vi "neuKLEIN.vi"() -> ()   [LabVIEW 2016] (continued)
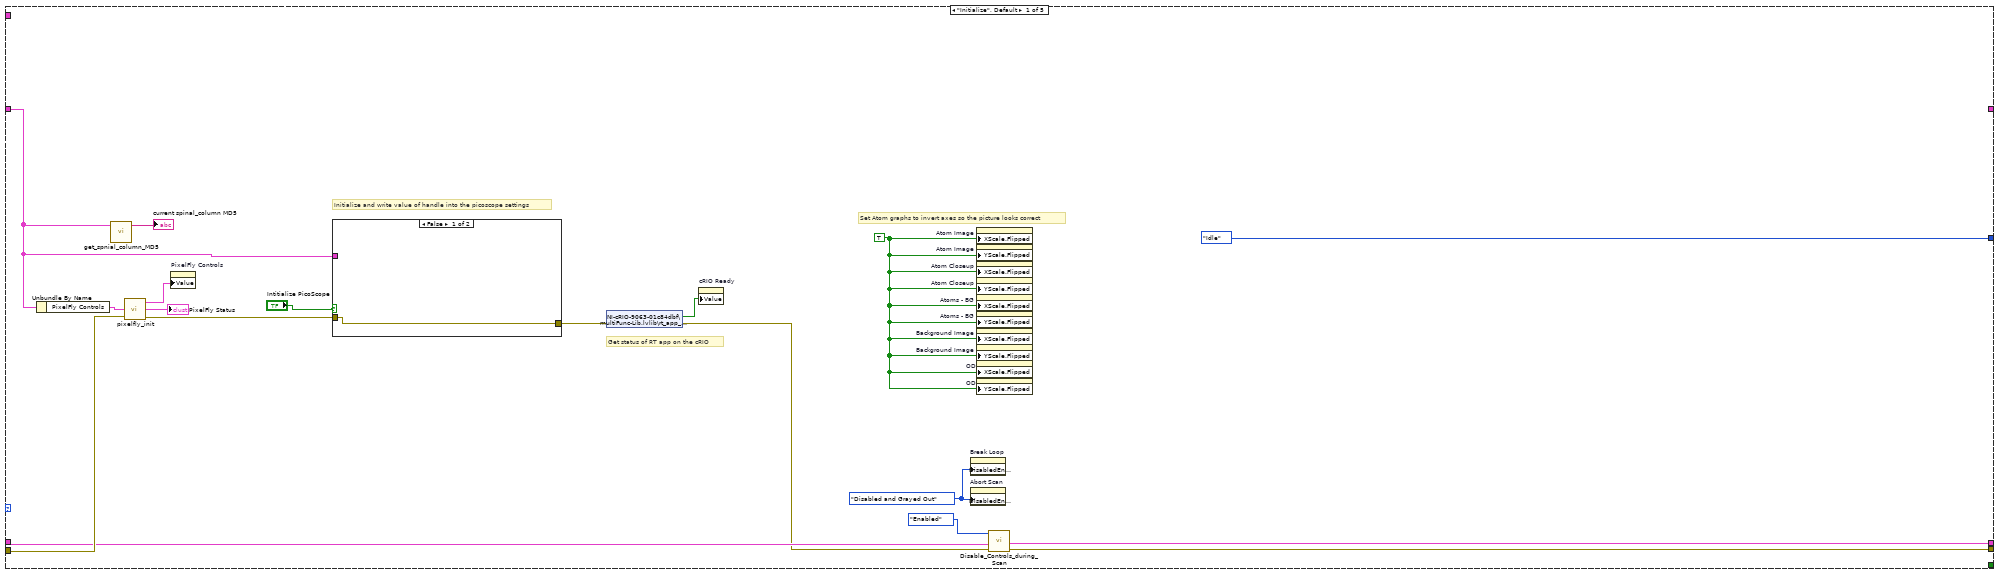
[diagram p2: hidden frame]
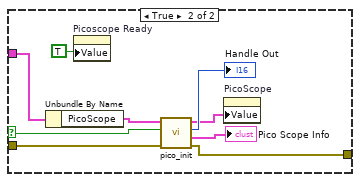
[diagram p3: hidden frame]
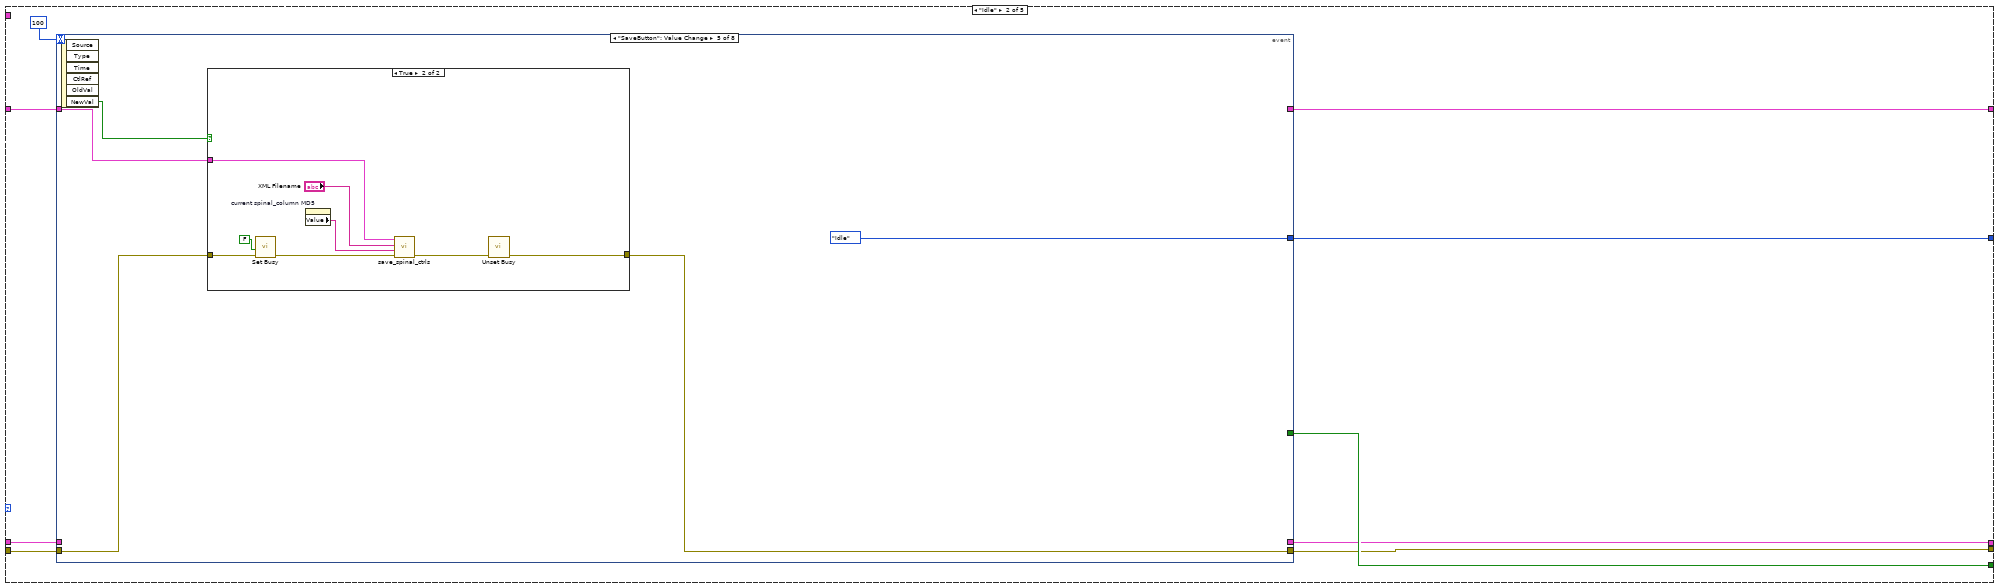
[diagram p4: hidden frame]
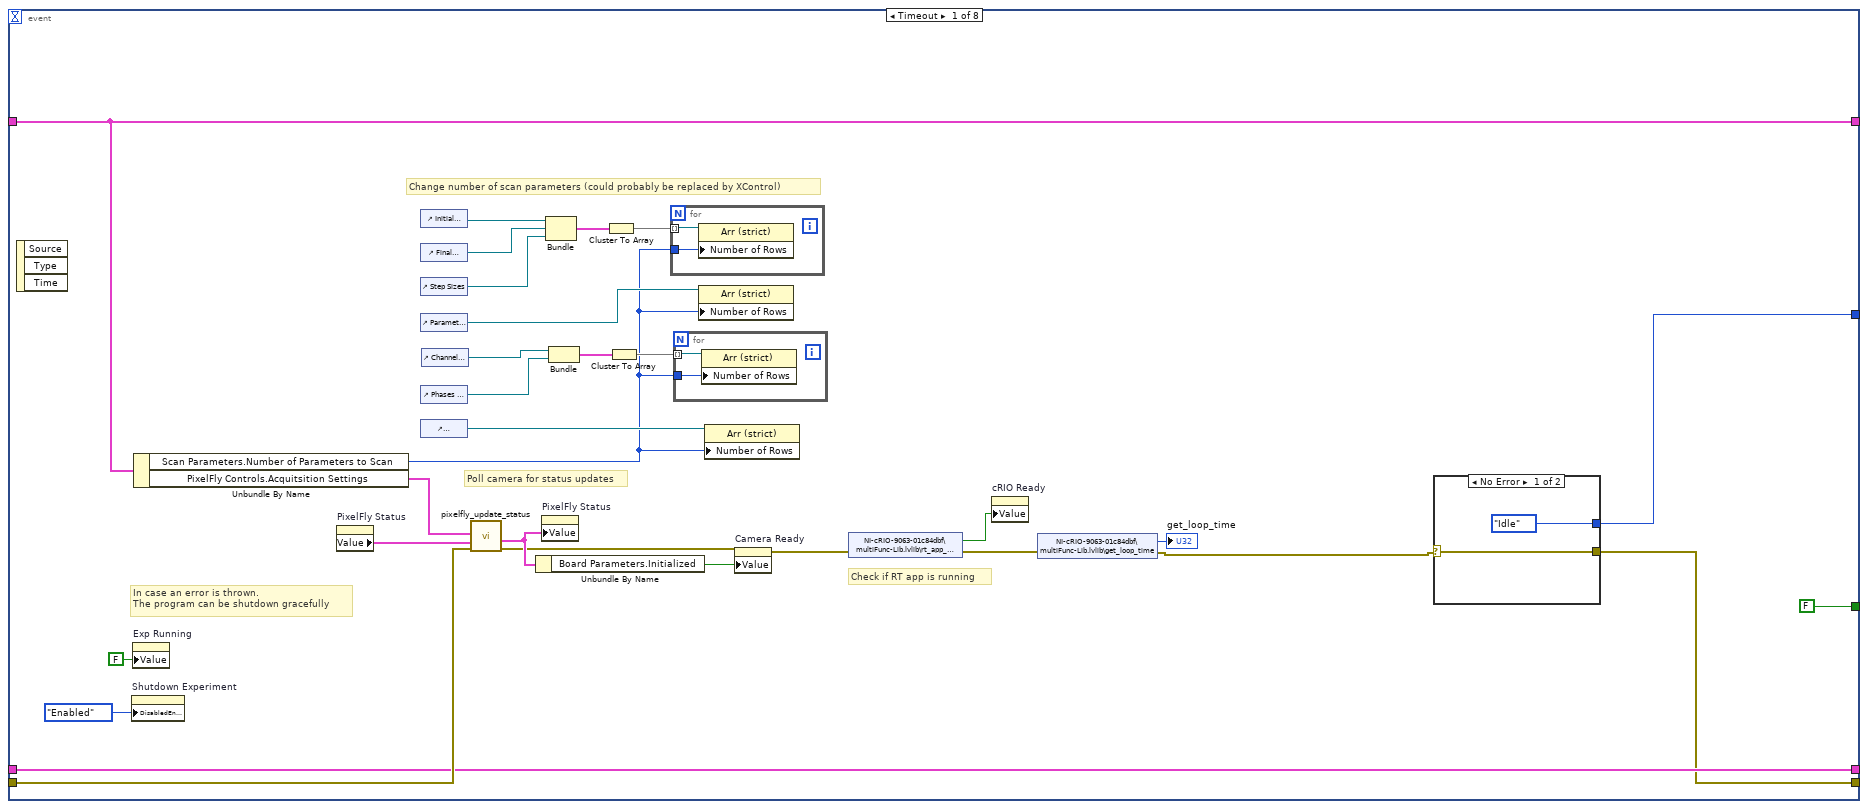
[diagram p5: hidden frame]
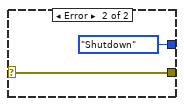
[diagram p6: hidden frame]
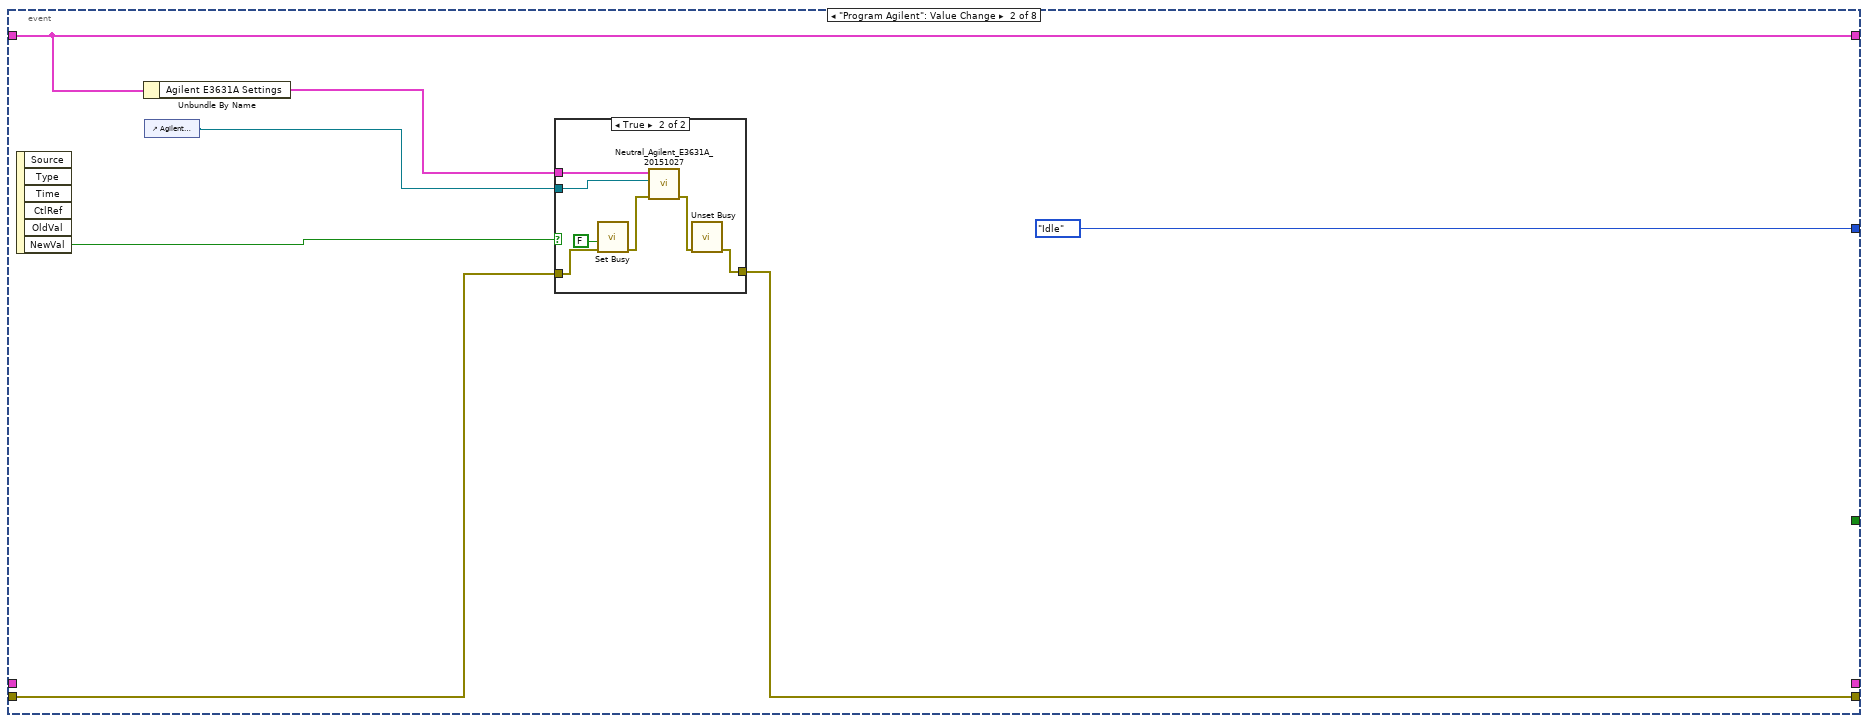
[diagram p7: hidden frame]
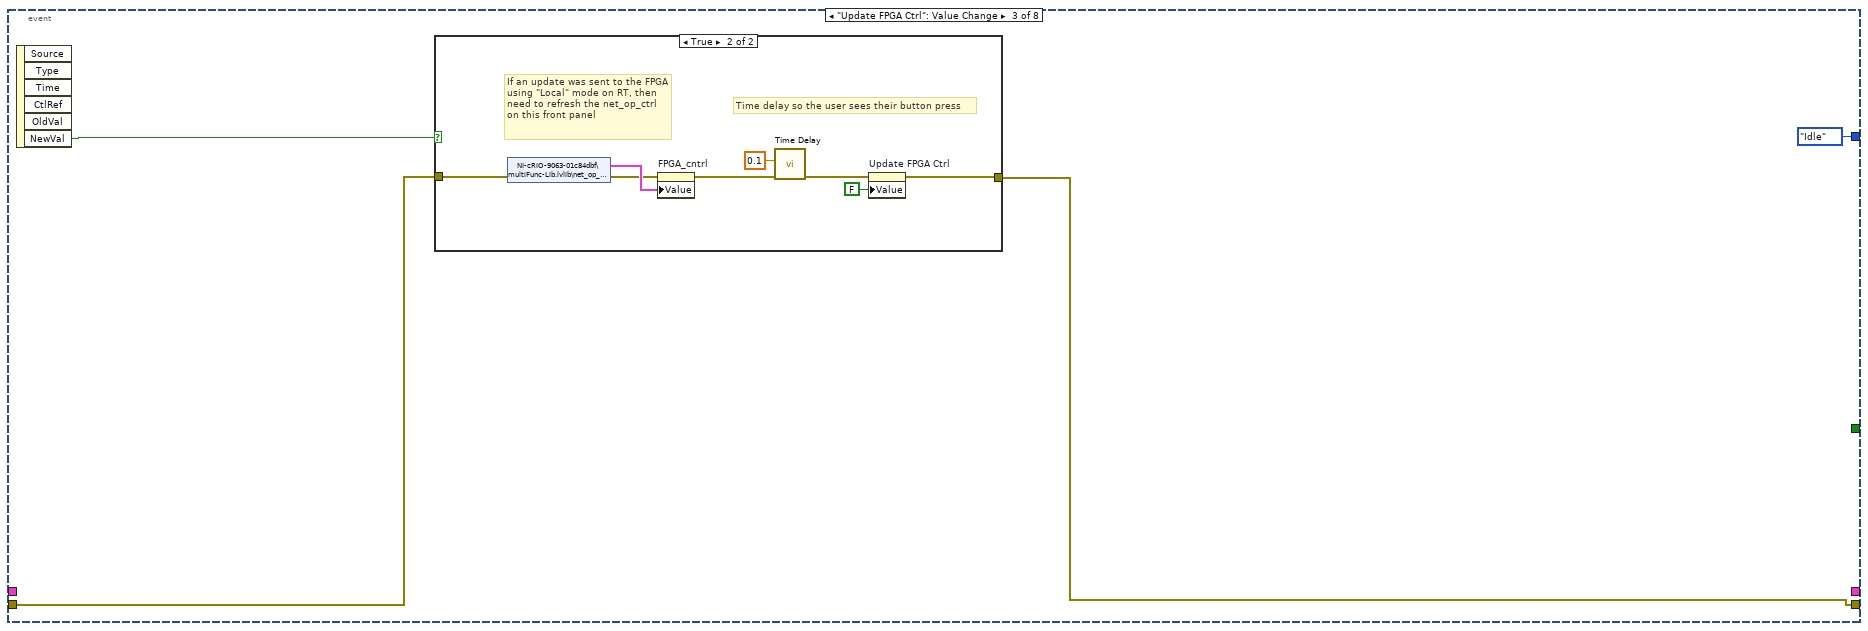
[diagram p9: hidden frame]
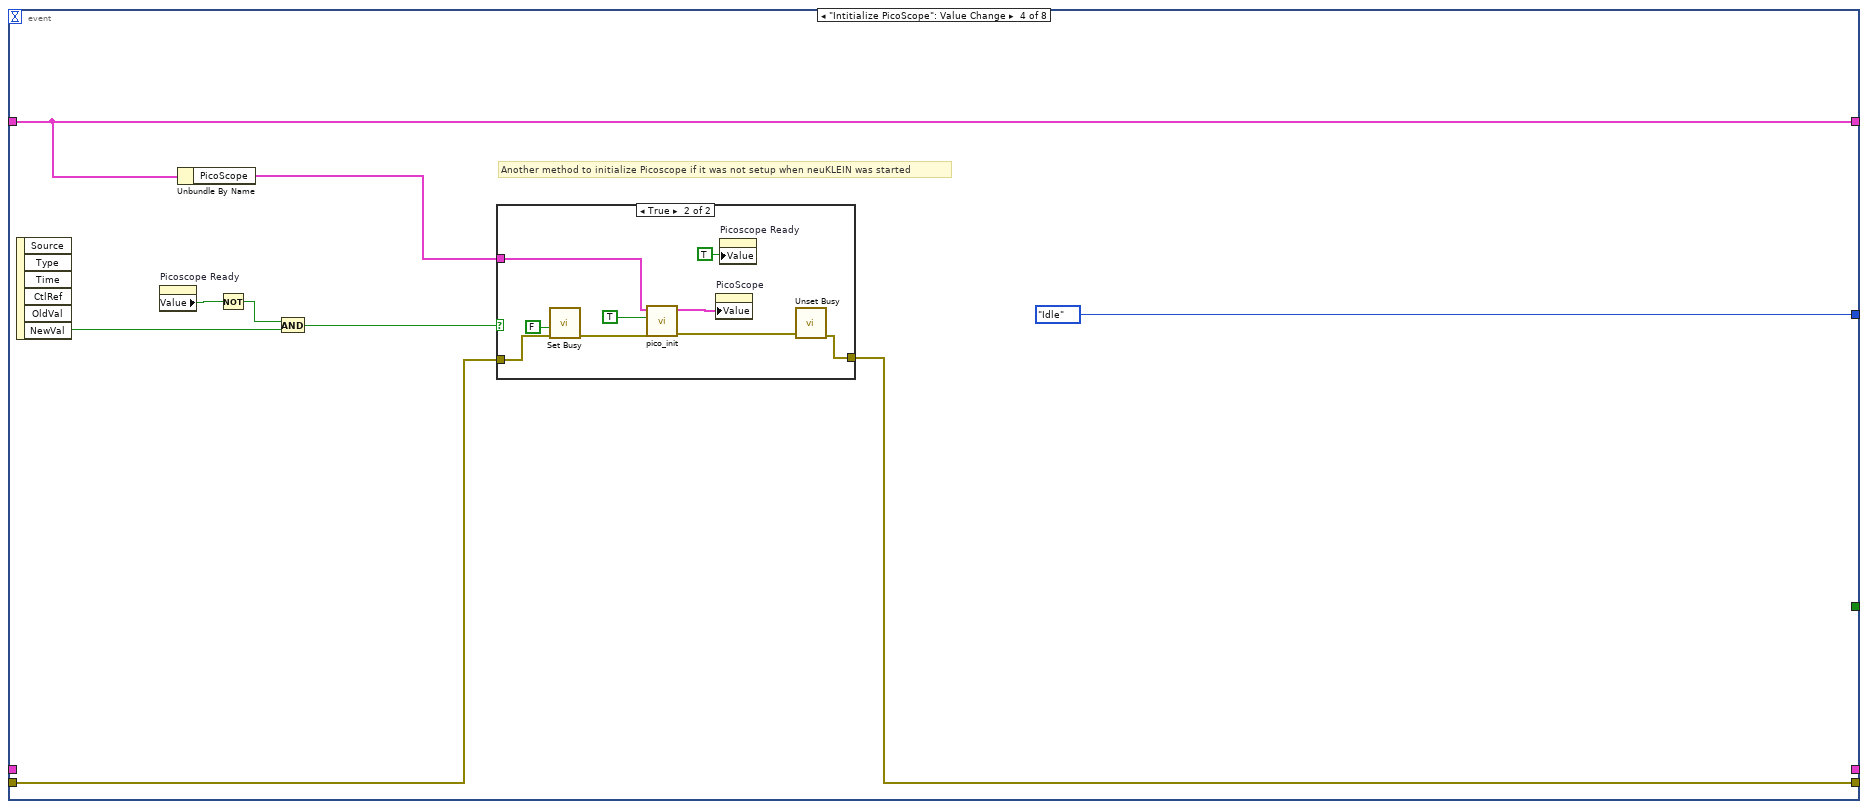
[diagram p11: hidden frame]
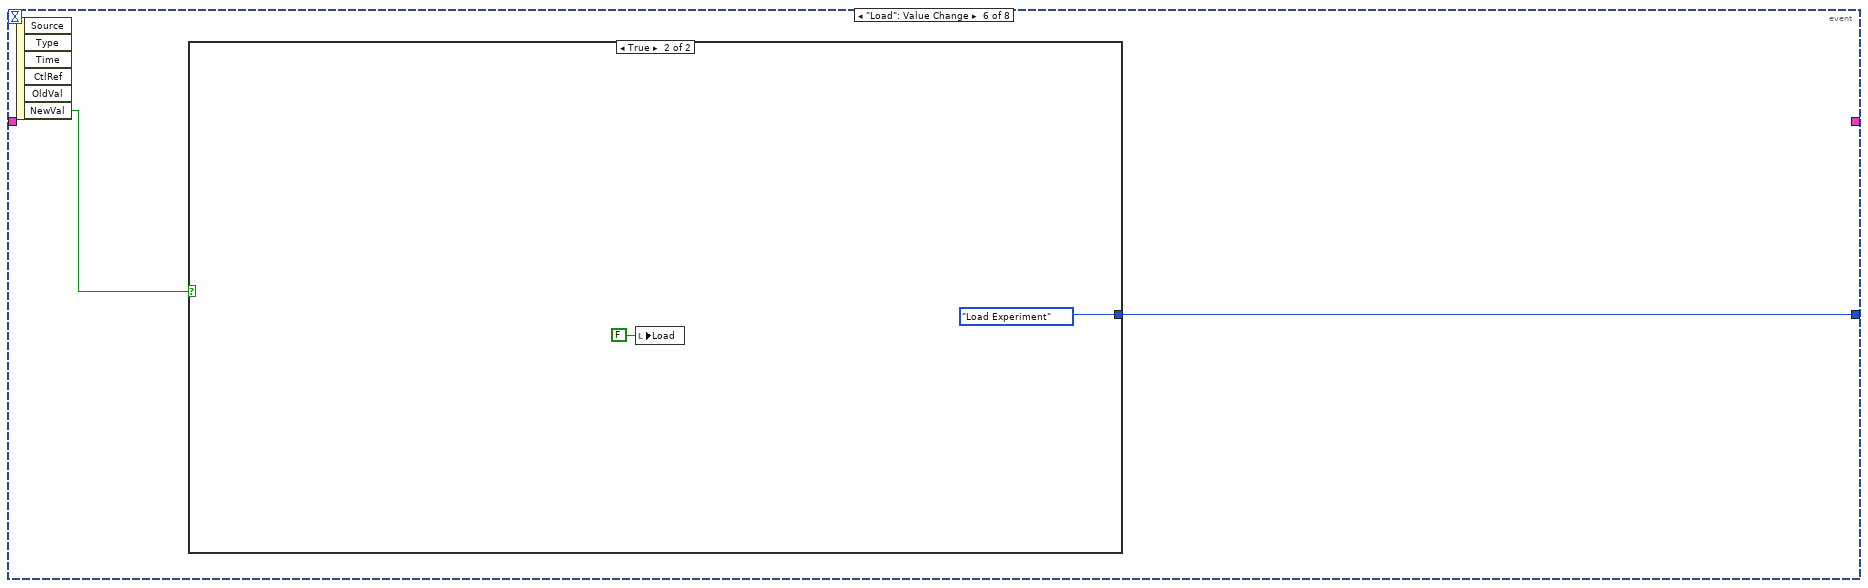
[diagram p14: hidden frame]
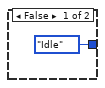
[diagram p15: hidden frame]
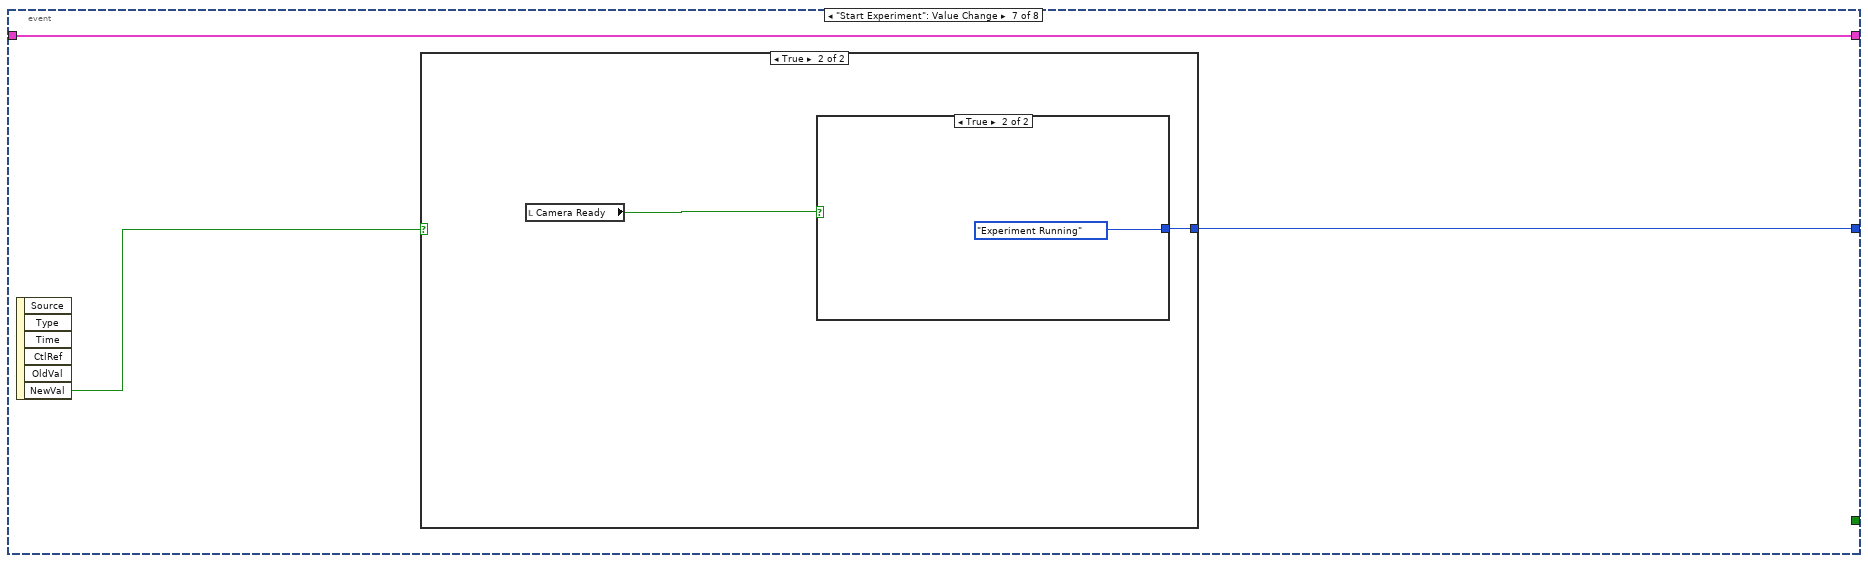
[diagram p16: hidden frame]
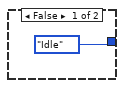
[diagram p17: hidden frame]
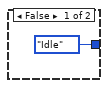
[diagram p18: hidden frame]
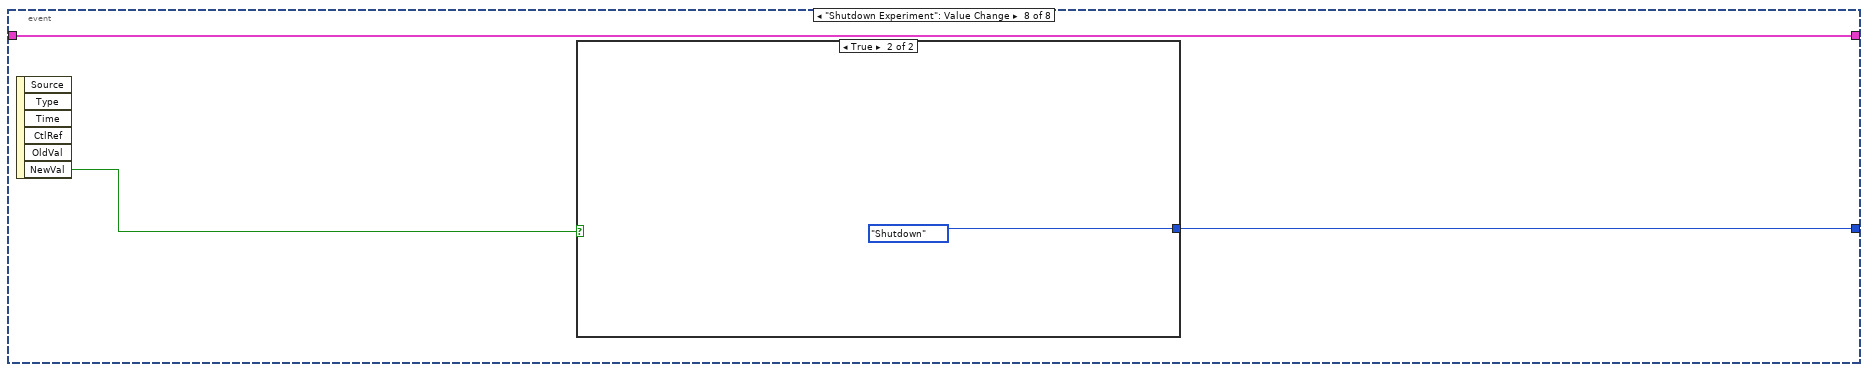
[diagram p19: hidden frame]
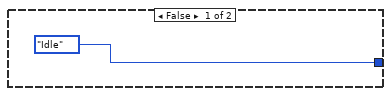
[diagram p20: hidden frame]
              frame False {
              }
              frame True {
                n79 = call <vilib>:"Set Busy.vi"("error in (no error)"=w147, "disable click? (T)"=FALSE) -> ("error out"=w144:errorcluster)  [unwired: 8 in, 1 out]
                n80 = call "pico_init.vi"("error in (no error)"=w144, "Initialize PicoScope?"=TRUE, "PicoScope Acquisition Settings Input"=w142) -> ("error out"=w143:errorcluster, "PicoScope Acquisition Settings Output"=w140:T39)  [unwired: 4 in, 2 out]
                n81 = property on="PicoScope" class="Clust (strict)"("Value"=w140) -> ()  [unwired: 2 in, 2 out]
                n82 = property on="Picoscope Ready" class="Bool (strict)"("Value"=TRUE ("Picoscope Ready")) -> ()  [unwired: 2 in, 2 out]
                n83 = call <vilib>:"Unset Busy.vi"("error in (no error)"=w143) -> ("error out"=w146:errorcluster)  [unwired: 10 in]
              }
            }
          }
          event "SaveButton": Value Change {
            n84 = event-data() -> ("NewVal"=w152:bool)  [unwired: 1 in, 5 out]
            n85 = case shown="True" w152 {
              tunnel: w151 -> [_ w156]
              tunnel: w149 -> [w153 w160]
              tunnel: [w153 w159] -> w148
              frame False {
              }
              frame True {
                n86 = call <vilib>:"Set Busy.vi"("error in (no error)"=w160, "disable click? (T)"=FALSE) -> ("error out"=w158:errorcluster)  [unwired: 8 in, 1 out]
                n87 = property on="current spinal_column MD5" class="Str"() -> ("Value"=w154:string)  [unwired: 2 in, 2 out]
                n88 = call "save_spinal_ctrls.vi"("error in (no error)"=w158, "MD5"=w154, "Name for file"="XML Filename", "spinal_column"=w156) -> ("error out"=w157:errorcluster)  [unwired: 5 in, 2 out]
                n89 = call <vilib>:"Unset Busy.vi"("error in (no error)"=w157) -> ("error out"=w159:errorcluster)  [unwired: 10 in]
              }
            }
          }
          event "Load": Value Change {
            n90 = event-data() -> ("NewVal"=w163:bool)  [unwired: 1 in, 5 out]
            n91 = case shown="True" w163 {
              tunnel: [rydberg_state_machine_states."Idle" rydberg_state_machine_states."Load Experiment"] -> w162
              frame False {
              }
              frame True {
                n92 = local write "Load"(FALSE ("Load")) -> ()
              }
            }
          }
          event "Start Experiment": Value Change {
            n93 = event-data() -> ("NewVal"=w169:bool)  [unwired: 1 in, 5 out]
            n94 = case shown="True" w169 {
              tunnel: [rydberg_state_machine_states."Idle" w172] -> w168
              frame False {
              }
              frame True {
                n95 = local read "Camera Ready"() -> (w171:bool)
                n96 = case shown="True" w171 {
                  tunnel: [rydberg_state_machine_states."Idle" rydberg_state_machine_states."Experiment Running"] -> w172
                  frame False {
                  }
                  frame True {
                  }
                }
              }
            }
          }
          event "Shutdown Experiment": Value Change {
            n97 = event-data() -> ("NewVal"=w177:bool)  [unwired: 1 in, 5 out]
            n98 = case shown="True" w177 {
              tunnel: [rydberg_state_machine_states."Idle" rydberg_state_machine_states."Shutdown"] -> w176
              frame False {
              }
              frame True {
              }
            }
          }
        }
      }
      frame "Experiment Running" {
        w180 = T62 3 items=["no dialog", "OK message", "continue or stop message", "OK message + warnings", "continue/stop + warnings"] ("type of dialog (OK msg:1)")
        # "Open Atom Shutter"
        # "Continue Exp. Running state if not aborted,\nno error, and Trigger Snap true"
        n99 = Unbundle By Name(w188) -> ("Scan Parameters"=w187:T5)
        n100 = property on="Trigger Snap Mode" class="Bool (strict)"() -> ("Value"=w190:bool)  [unwired: 2 in, 2 out]
        n101 = Get Date/Time In Seconds() -> (seconds since 1Jan1904=w204:timestamp)
        n102 = local write "Exp Running"(TRUE) -> ()
        n103 = local write "Start Experiment"(FALSE ("Start Experiment")) -> ()
        n104 = call "calculate_parameters.vi"("Experimental Variables"=w196) -> ("Calculated Experimental Values"=→"Calculated Experimental Values":T10)  [unwired: 8 in, 2 out]
        n105 = call "Disable_Controls_during_Scan.vi"("Error In"=w203, "Control Reference Cluster Input"=w191, "Control State In"=T58."Disabled and Grayed Out" ("Disabled")) -> ("error out"=w194:errorcluster, "Control Reference Cluster Output"=w201:T56)  [unwired: 7 in]
        n106 = property on="Abort Scan" class="Bool (strict)"("DisabledEnum"=T58."Enabled" ("Disabled")) -> ()  [unwired: 2 in, 2 out]
        n107 = call "GenerateScanArrays.vi"("time stamp"=w204, "In Trigger Snap Mode?"=w190, "Scan Parameters"=w187) -> ("Parameter Array"=w192:dbl[][], "Array"=w195:dbl[])  [unwired: 6 in, 1 out]
        n108 = call "Progress Bar Initialization.vi"("Array"=w192, "Trigger Snap or Scan?"=w190, "error in (no error)"=w194) -> ("Scan Progress"=w186:T49, "error out"=w193:errorcluster)  [unwired: 6 in]
        n109 = call "atomShutterCtrl.vi"("Atom Shutter"=TRUE) -> ()
        n110 = property on="Scan Progress" class="Clust (strict)"("Value"=w186) -> ()  [unwired: 2 in, 2 out]
        n111 = for {
          tunnel: w190 -> [w258]
          shift-right: [w232] -> _
          shift-left: w188 -> [w231]
          shift-right: [w238] -> w185
          shift-left: w193 -> [w271]
          tunnel: w192 -> [w260] mode=indexing
          tunnel: w195 -> [w255]
          tunnel: w204 -> [w253]
          tunnel: w201 -> [w245]
          tunnel: [w245] -> w200
          tunnel: w196 -> [w247]
          tunnel: ["Abort Scan"] -> w183
          i -> [w246]
          stop <- "Abort Scan" stop-if-true
          # "This is going to execute at the beginning of the loop.\nWill try to fix it when I get aruond to implementing a\nfull state machine"
          # "Allows for scans to be aborted"
          n112 = call "Change_ParameterV2.vi"("Started In Trig Snap?"=w258, "Parameter Values In"=w260, "Spinal Column In"=w231) -> ("Current Parameter Values"=w254:dbl[], "Spinal Column Out"=w259:T63)  [unwired: 7 in]
          "Current Param. Values" <- w254
          n113 = property on="Take Pictures" class="Bool (strict)"() -> ("Value"=w234:bool)  [unwired: 2 in, 2 out]
          n114 = call "WriteExp.vi"("error in (no error)"=w271, "Take Pictures"=w234, "Spinal Column In"=w259) -> ("error out"=w249:errorcluster, "Spinal Column Out"=w263:T63)  [unwired: 7 in]
          n115 = call "DoExperiment.vi"("Spinal Column In"=w263, "Take Pictures"=w234, "Error In"=w249) -> ("error out"=w238:errorcluster, "Channel B Out"=w243:dbl[][][], "Channel A Out"=w242:dbl[][][], "Spinal Column Out"=w250:T63, "Atom Image"=w270:dbl[][], "Background Image"=w269:dbl[][], "Buffer status"=→"Buffer status":T14, "Wavemeter"=w233:string)  [unwired: 9 in]
          "Wavemeter" <- w233
          n116 = call "rapid_xy.vi"("Channel A Out"=w242) -> ("xy array"=→"Pico Scope Channel A":T53)  [unwired: 10 in]
          n117 = call "rapid_xy.vi"("Channel A Out"=w243) -> ("xy array"=→"Pico Scope Channel B":T53)  [unwired: 10 in]
          n118 = call "BG_Subtraction.vi"("Background Image"=w269, "Atom Image"=w270) -> ("Background Image Out"=w257:dbl[][], "Atom Image Out"=w265:dbl[][], "Atoms - BG"=w266:dbl[][])  [unwired: 7 in]
          "Atom Image" <- w265
          "Background Image" <- w257
          "Atoms - BG" <- w266
          n119 = property on="Atoms - BG" class="IntGraph (strict)"() -> ("CrsrLis"=w267:T64)  [unwired: 2 in, 2 out]
          n120 = call "CutIMG.vi"("Full Image In"=w266, "Cursor List"=w267) -> ("Cut Image Out"=→"Atom Closeup":dbl[][])  [unwired: 9 in]
          n121 = case shown="\"Fancy\"" "Set Analysis Mode" {
            tunnel: w267 -> [w282 w296]
            tunnel: w265 -> [w281 w295]
            tunnel: w257 -> [w280 w294]
            tunnel: [w279 w293] -> w256
            tunnel: [w278 w291] -> w228
            tunnel: [w273 w290] -> w241
            tunnel: [w276 w289] -> w236
            tunnel: [w276 w288] -> w235
            tunnel: w247 -> [w277 w287]
            tunnel: [T52 {"Amplitude (OD)"=0.0, "X Center (px)"=0.0, "Y Center (px)"=0.0, " X Width (um)"=0.0, "Y Width (um)"=0.0, "Aspect Ratio"=0.0, "Rot. Angle (deg)"=0.0} ("Best Fit Parameter Cluster") w286] -> w240
            tunnel: [u32 0 ("Elapsed time ( ms)") w285] -> w239
            tunnel: [0.0 ("Phase Space Density") w284] -> w237
            frame "Fast", Default {
              w276 = 1.0 ("Temperature (K) x")
              n122 = call "CountAtomsFast.vi"("Experimental Variables"=w277, "Background Image"=w280, "Atom Image"=w281, "Cursor List"=w282) -> ("Data Cuts"=w273:dbl[][], "OD"=w279:dbl[][], "Number"=w278:dbl)  [unwired: 5 in]
            }
            frame "Fancy" {
              n123 = call "CountAtoms_LVFitting.vi"("Cursor List"=w296, "Atom Image"=w295, "Experimental Variables"=w287, "Background Image"=w294, "Drop Time"="Drop Time", "Trap Frequencies"="Trap Frequencies") -> ("Elapsed time ( ms)"=w285:u32, "Number"=w291:dbl, "OD"=w293:dbl[][], "Data Cuts"=w290:dbl[][], "Temperature (K) x"=w289:dbl, "Phase Space Density"=w284:dbl, "Best Fit Parameter Cluster"=w286:T52, "Temperature (K) y"=w288:dbl)  [unwired: 1 in, 1 out]
            }
          }
          "GIANT Atoms" <- w256
          "OD" <- w256
          "Number" <- w228
          "Atom Number Chart" <- w228
          "Temp. (K) - Y" <- w235
          "Temp. (K) - X" <- w236
          "Giant Data Cuts" <- w241
          "Data Cuts" <- w241
          "Best Fit Parameter Cluster" <- w240
          "Elapsed time ( ms)" <- w239
          "Phase Space Density" <- w237
          n124 = property on="Atom Number Chart" class="WFChart (strict)"() -> ("XScale.Maximum"=w225:dbl)  [unwired: 2 in, 2 out]
          n125 = property on="Atom Number Chart" class="WFChart (strict)"() -> ("History Data"=w224:dbl[])  [unwired: 2 in, 2 out]
          n126 = property on="Temperature Chart" class="WFChart (strict)"() -> ("History Data"=w223:T65)  [unwired: 2 in, 2 out]
          n127 = Bundle("Temperature (K) x"=w236, "Temperature (K) y"=w235) -> (→"Temperature Chart":T51)  [unwired: 1 in]
          n128 = Bundle(cluster="output cluster", "Number"=w228, "OD"=w256, "Data Cuts"=w241, "Temperature (K) x"=w236, "Temperature (K) y"=w235) -> (w252:T46)
          n129 = case shown="False" w258 {
            tunnel: w270 -> [w312 _]
            tunnel: w269 -> [w311 _]
            tunnel: w243 -> [w310 _]
            tunnel: w242 -> [w309 _]
            tunnel: w255 -> [w308 _]
            tunnel: w246 -> [w299 _]
            tunnel: w254 -> [w307 _]
            tunnel: w253 -> [w306 _]
            tunnel: w250 -> [w305 w313]
            tunnel: w252 -> [w304 _]
            tunnel: [w300 w313] -> w232
            tunnel: w233 -> [w297 _]
            frame False {
              # "Increment progress bar"
              n130 = Increment(x=w299) -> (x+1=w298:i32)
              n131 = property on="Current Pnt Num" class="DigNum (strict)"("Value"=w298) -> ()  [unwired: 2 in, 2 out]
              n132 = call "GenerateBatchFilesV2.vi"("Spinal Column In"=w305, "output cluster"=w304, "time stamp"=w306, "Current Values"=w307, "Loop Iteration"=w299, "Wavemeter"=w297, "Independent Variable Array"=w308) -> ("Scan Parameters.Raw_Data Folder"=w303:path, "Spinal Column Out"=w300:T63, "Full Scan Name Out"=w301:string, "Image Number"=w302:i32)  [unwired: 3 in, 2 out]
              "Scan Name" <- w301
              n133 = call "SaveImages.vi"("Background Image In"=w311, "Atoms Image In"=w312, "Base Filename"=w301, "Raw Data Path"=w303, "ImageNumber"=w302) -> ()  [unwired: 9 in, 2 out]
              n134 = call "save_pico_data.vi"("full scan name"=w301, "Img #"=w302, "Channel B In"=w310, "Channel A In"=w309, "Spinal Column In"=w300) -> ()  [unwired: 7 in]
            }
            frame True {
            }
          }
          n135 = Bundle("XScale.Maximum"=w225, "History Data"=w224, "History Data"=w223) -> (w222:T66)  [unwired: 1 in]
          n136 = call "numAndTempStats.vi"("Stat. Limits"="Stat. Limits", "Stats Flag"="Stats Flag", "strip chart properties"=w222) -> ("Num and Temp Stats"=→"Num and Temp Stats":T47)  [unwired: 8 in]
        }
        n137 = property on="Trigger Snap Mode" class="Bool (strict)"() -> ("Value"=w184:bool)  [unwired: 2 in, 2 out]
        n138 = Compound Arithmetic op=AND(invert w183, w184, invert w185) -> (w182:bool)
        n139 = case shown="False" w182 {
          tunnel: [rydberg_state_machine_states."Idle" rydberg_state_machine_states."Experiment Running"] -> w207
          tunnel: w185 -> [w215 w219]
          tunnel: [w214 w219] -> w181
          tunnel: w200 -> [w212 w220]
          tunnel: [w211 w220] -> w199
          frame False {
            # "Close Atom Shutter"
            # "Reset abort button if pressed"
            n140 = property on="Abort Scan" class="Bool (strict)"() -> ("Value"=w210:bool)  [unwired: 2 in, 2 out]
            n141 = case shown="True" w210 {
              frame False {
              }
              frame True {
                # "Reset this in case it is true"
                n142 = property on="Abort Scan" class="Bool (strict)"("Value"=FALSE) -> ()  [unwired: 2 in, 2 out]
                n143 = property on="Trigger Snap Mode" class="Bool (strict)"("Value"=FALSE ("Trigger Snap Mode")) -> ()  [unwired: 2 in, 2 out]
              }
            }
            n144 = property on="Abort Scan" class="Bool (strict)"("DisabledEnum"=T58."Disabled and Grayed Out" ("Disabled")) -> ()  [unwired: 2 in, 2 out]
            n145 = call "atomShutterCtrl.vi"("Atom Shutter"=FALSE) -> ()
            n146 = call "Disable_Controls_during_Scan.vi"("Error In"=w215, "Control Reference Cluster Input"=w212, "Control State In"=T58."Enabled" ("Disabled")) -> ("error out"=w214:errorcluster, "Control Reference Cluster Output"=w211:T56)  [unwired: 7 in]
          }
          frame True {
          }
        }
        n147 = call <vilib>:"Simple Error Handler.vi"("type of dialog (OK msg:1)"=w180, "error in (no error)"=w181) -> ()  [unwired: 3 in, 5 out]
      }
      frame "Load Experiment" {
        n148 = property on="current spinal_column MD5" class="Str"() -> ("Value"=w314:string)  [unwired: 2 in, 2 out]
        n149 = call <vilib>:"Set Busy.vi"("error in (no error)"=w323, "disable click? (T)"=FALSE) -> ("error out"=w317:errorcluster)  [unwired: 8 in, 1 out]
        n150 = call "load_spinal_ctrls.vi"("spinal_column"=w316, "MD5"=w314, "DAT File Location"="XML File Location", "error in (no error)"=w317) -> ("Spinal Column Out"=w319:T63, "error out"=w318:errorcluster)  [unwired: 4 in]
        n151 = call <vilib>:"Unset Busy.vi"("error in (no error)"=w318) -> ("error out"=w322:errorcluster)  [unwired: 10 in]
        n152 = Unbundle By Name(w319) -> ("48ch_pb_array"=w321:T3, "Red MOT 87 Inputs"=w335:T21, "ODT Params"=w333:T25, "Red MOT 88 Inputs"=w332:T21, "Agilent E3631A Settings"=w327:T43, "Scan Parameters"=w331:T5, "PicoScope"=w330:T39, "6713 Blue MOT"=w329:T16, "6229 Green Lattice Inputs"=w328:T28, "Novatech Synth Settings"=w325:T36[][], "FPGA_cntrl"=w320:T30)
        n153 = property on="48ch_pb_array" class="Arr (strict)"("Value"=w321) -> ()  [unwired: 2 in, 2 out]
        n154 = property on="Red MOT 87 Inputs" class="Clust (strict)"("Value"=w335) -> ()  [unwired: 2 in, 2 out]
        n155 = property on="ODT Params" class="Clust (strict)"("Value"=w333) -> ()  [unwired: 2 in, 2 out]
        n156 = property on="Red MOT 88 Inputs" class="Clust (strict)"("Value"=w332) -> ()  [unwired: 2 in, 2 out]
        n157 = property on="Agilent E3631A Settings" class="Clust (strict)"("Value"=w327) -> ()  [unwired: 2 in, 2 out]
        n158 = property on="Scan Parameters" class="Clust (strict)"("Value"=w331) -> ()  [unwired: 2 in, 2 out]
        n159 = property on="PicoScope" class="Clust (strict)"("Value"=w330) -> ()  [unwired: 2 in, 2 out]
        n160 = property on="6713 Blue MOT" class="Clust (strict)"("Value"=w329) -> ()  [unwired: 2 in, 2 out]
        n161 = property on="6229 Green Lattice Inputs" class="Clust (strict)"("Value"=w328) -> ()  [unwired: 2 in, 2 out]
        n162 = property on="Novatech Synth Settings" class="Arr (strict)"("Value"=w325) -> ()  [unwired: 2 in, 2 out]
        n163 = property on="FPGA_cntrl" class="Clust (strict)"("Value"=w320) -> ()  [unwired: 2 in, 2 out]
      }
      frame "Shutdown" {
        w336 = FALSE ("Value")
        # "Close Atom Shutter\nJust in case"
        n164 = call "atomShutterCtrl.vi"("Atom Shutter"=FALSE) -> ()
        n165 = local write "Shutdown Experiment"(FALSE ("Shutdown Experiment")) -> ()
        n166 = property on="Initialized" class="Bool (strict)"(error in=w344, "Value"=w336) -> (error out=w342:errorcluster)  [unwired: 1 in, 1 out]
        n167 = property on="Running" class="Bool (strict)"(error in=w342, "Value"=w336) -> (error out=w341:errorcluster)  [unwired: 1 in, 1 out]
        n168 = Unbundle By Name(w348) -> ("PicoScope.Pico Scope Inititalization Settings.Handle"=w347:i16, "PixelFly Controls.Acquitsition Settings"=w346:T12)
        n169 = property on="Camera Ready" class="Bool (strict)"(error in=w341, "Value"=w336) -> (error out=w340:errorcluster)  [unwired: 1 in, 1 out]
        n170 = property on="Picoscope Ready" class="Bool (strict)"(error in=w340, "Value"=w336) -> (error out=w339:errorcluster)  [unwired: 1 in, 1 out]
        n171 = property on="Intitialize PicoScope" class="Bool (strict)"(error in=w339, "Value"=w336) -> (error out=w338:errorcluster)  [unwired: 1 in, 1 out]
        n172 = property on="Use PicoScope?" class="Bool (strict)"(error in=w338, "Value"=w336) -> (error out=w337:errorcluster)  [unwired: 1 in, 1 out]
        n173 = property on="cRIO Ready" class="Bool (strict)"(error in=w337, "Value"=w336) -> (error out=w343:errorcluster)  [unwired: 1 in, 1 out]
        n174 = call "pixelfly_close.vi"("error in (no error)"=w343, "Acquitsition Settings"=w346) -> ("error out"=w345:errorcluster)  [unwired: 2 in]
        n175 = call "PicoScope5000aClose.vi"("error in (no error)"=w345, "handle"=w347) -> ("error out"=w351:errorcluster)  [unwired: 1 in]
      }
    }
    "error out" <- w7
  }
